vi "Dresden R2R Sputter 03.02.2018 IY24.vi"() -> ()   [LabVIEW 2009] (continued)
                                n22000 = Or(x=w22962, y=w22961) -> (x .or. y?=w22960:bool)
                                }
                                }
                                frame #1 {
                                }
                                }
                                }
                                frame #1 {
                                n22001 = local read "Semi"() -> (w22973:bool)
                                n22002 = case shown="False" w22973 {
                                frame #0 {
                                n22003 = Wait Until Next ms Multiple(millisecond multiple=u32 1000) -> ()  [unwired: 1 out]
                                n22004 = local write "Ch4_PA22"(TRUE ("PA3")) -> ()
                                }
                                frame #1 {
                                }
                                }
                                }
                                }
                              }
                              frame #1 {
                              }
                            }
                          }
                          frame #18 {
                            # "START MP"
                            n22005 = local read "Semi"() -> (w22976:bool)
                            n22006 = case shown="False" w22976 {
                              frame #0 {
                                n22007 = stacked-sequence {
                                frame #0 {
                                n22008 = local read "Semi"() -> (w22977:bool)
                                n22009 = case shown="False" w22977 {
                                frame #0 {
                                n22010 = while {
                                i -> [w22984]
                                stop <- w22978 stop-if-true
                                n22011 = Greater?(x=w22984, y=50) -> (0:w22982:bool)
                                n22012 = case shown="True" w22982 {
                                frame #0 {
                                }
                                frame #1 {
                                n22013 = local write "Semi"(TRUE ("Semi")) -> ()
                                n22014 = local write "Error Message"("Start up process  cancelled\nbecause MP4 not started.\nPlease check MP4 connections." ("Error Message")) -> ()
                                }
                                }
                                n22015 = local read "Ch4_Mp_di"() -> (w22981:bool)
                                n22016 = case shown="False" w22981 {
                                tunnel: [FALSE TRUE] -> w22980
                                frame #0 {
                                n22017 = Wait Until Next ms Multiple(millisecond multiple=u32 200) -> ()  [unwired: 1 out]
                                n22018 = local write "Ch4_Mp_do"(TRUE ("Ch1_Tp_bv_do")) -> ()
                                }
                                frame #1 {
                                }
                                }
                                n22019 = local read "Semi"() -> (w22979:bool)
                                n22020 = Or(x=w22980, y=w22979) -> (x .or. y?=w22978:bool)
                                }
                                }
                                frame #1 {
                                }
                                }
                                }
                                frame #1 {
                                n22021 = local read "Semi"() -> (w22991:bool)
                                n22022 = case shown="False" w22991 {
                                frame #0 {
                                n22023 = local write "Ch4_PA25"(TRUE ("PA3")) -> ()
                                n22024 = Wait Until Next ms Multiple(millisecond multiple=u32 1000) -> ()  [unwired: 1 out]
                                }
                                frame #1 {
                                }
                                }
                                }
                                }
                              }
                              frame #1 {
                              }
                            }
                          }
                          frame #19 {
                            # "CHECK PL-PRESSURE"
                            n22025 = local read "Semi"() -> (w22994:bool)
                            n22026 = case shown="False" w22994 {
                              frame #0 {
                                n22027 = stacked-sequence {
                                frame #0 {
                                n22028 = local read "Semi"() -> (w22995:bool)
                                n22029 = case shown="False" w22995 {
                                frame #0 {
                                n22030 = while {
                                i -> [w23004]
                                stop <- w22999 stop-if-true
                                n22031 = Greater?(x=w23004, y=1200) -> (0:w23002:bool)
                                n22032 = case shown="True" w23002 {
                                frame #0 {
                                }
                                frame #1 {
                                n22033 = local write "Semi"(TRUE ("Semi")) -> ()
                                n22034 = local write "Error Message"("Start up process was cancelled.\nPlease check Pipeline \nvacuum connections." ("Error Message")) -> ()
                                }
                                }
                                n22035 = local read "Pl_pg_press_ch4"() -> (w22998:dbl)
                                n22036 = Less?(x=w22998, y=0.9) -> (x < y?=w22996:bool)
                                n22037 = case shown="False" w22996 {
                                tunnel: [FALSE TRUE] -> w23001
                                frame #0 {
                                n22038 = Wait Until Next ms Multiple(millisecond multiple=u32 500) -> ()  [unwired: 1 out]
                                }
                                frame #1 {
                                }
                                }
                                n22039 = local read "Semi"() -> (w23000:bool)
                                n22040 = Or(x=w23001, y=w23000) -> (x .or. y?=w22999:bool)
                                }
                                }
                                frame #1 {
                                }
                                }
                                }
                                frame #1 {
                                n22041 = local read "Semi"() -> (w23010:bool)
                                n22042 = case shown="False" w23010 {
                                frame #0 {
                                n22043 = local write "Ch4_PA26"(TRUE ("PA3")) -> ()
                                n22044 = Wait Until Next ms Multiple(millisecond multiple=u32 1000) -> ()  [unwired: 1 out]
                                }
                                frame #1 {
                                }
                                }
                                }
                                }
                              }
                              frame #1 {
                              }
                            }
                          }
                          frame #20 {
                            # "START TP"
                            n22045 = local read "Semi"() -> (w23013:bool)
                            n22046 = case shown="False" w23013 {
                              frame #0 {
                                n22047 = stacked-sequence {
                                frame #0 {
                                n22048 = local read "Semi"() -> (w23014:bool)
                                n22049 = case shown="False" w23014 {
                                frame #0 {
                                n22050 = stacked-sequence {
                                frame #0 {
                                n22051 = local read "Semi"() -> (w23015:bool)
                                n22052 = case shown="False" w23015 {
                                frame #0 {
                                n22053 = local write "Tp4_auto_start"(TRUE ("Tp1_auto_start")) -> ()
                                }
                                frame #1 {
                                }
                                }
                                }
                                frame #1 {
                                n22054 = local read "Semi"() -> (w23017:bool)
                                n22055 = case shown="False" w23017 {
                                frame #0 {
                                n22056 = Wait (ms)(milliseconds to wait=u32 1000) -> ()  [unwired: 1 out]
                                }
                                frame #1 {
                                }
                                }
                                }
                                frame #2 {
                                n22057 = local read "Semi"() -> (w23019:bool)
                                n22058 = case shown="False" w23019 {
                                frame #0 {
                                n22059 = local write "Tp4_auto_start"(TRUE ("Tp1_auto_start")) -> ()
                                }
                                frame #1 {
                                }
                                }
                                }
                                }
                                }
                                frame #1 {
                                }
                                }
                                }
                                frame #1 {
                                n22060 = local read "Semi"() -> (w23021:bool)
                                n22061 = case shown="False" w23021 {
                                frame #0 {
                                n22062 = local write "Ch4_PA30"(TRUE ("PA3")) -> ()
                                n22063 = Wait Until Next ms Multiple(millisecond multiple=u32 1000) -> ()  [unwired: 1 out]
                                }
                                frame #1 {
                                }
                                }
                                }
                                }
                              }
                              frame #1 {
                              }
                            }
                          }
                          frame #21 {
                            # "CHECK CH-PRESSURE"
                            n22064 = local read "Semi"() -> (w23024:bool)
                            n22065 = case shown="False" w23024 {
                              frame #0 {
                                n22066 = stacked-sequence {
                                frame #0 {
                                n22067 = local read "Semi"() -> (w23025:bool)
                                n22068 = case shown="False" w23025 {
                                frame #0 {
                                n22069 = while {
                                i -> [w23034]
                                stop <- w23029 stop-if-true
                                n22070 = Greater?(x=w23034, y=1200) -> (0:w23032:bool)
                                n22071 = case shown="True" w23032 {
                                frame #0 {
                                }
                                frame #1 {
                                n22072 = local write "Semi"(TRUE ("Semi")) -> ()
                                n22073 = local write "Error Message"("Start up process was cancelled.\nPlease check chamber \nvacuum connections." ("Error Message")) -> ()
                                }
                                }
                                n22074 = local read "Ch4pressure"() -> (w23028:dbl)
                                n22075 = Less?(x=w23028, y=0.9) -> (x < y?=w23026:bool)
                                n22076 = case shown="False" w23026 {
                                tunnel: [FALSE TRUE] -> w23031
                                frame #0 {
                                n22077 = Wait Until Next ms Multiple(millisecond multiple=u32 500) -> ()  [unwired: 1 out]
                                }
                                frame #1 {
                                }
                                }
                                n22078 = local read "Semi"() -> (w23030:bool)
                                n22079 = Or(x=w23031, y=w23030) -> (x .or. y?=w23029:bool)
                                }
                                }
                                frame #1 {
                                }
                                }
                                }
                                frame #1 {
                                n22080 = local read "Semi"() -> (w23040:bool)
                                n22081 = case shown="False" w23040 {
                                frame #0 {
                                n22082 = local write "Ch4_PA27"(TRUE ("PA3")) -> ()
                                n22083 = Wait Until Next ms Multiple(millisecond multiple=u32 1000) -> ()  [unwired: 1 out]
                                }
                                frame #1 {
                                }
                                }
                                }
                                }
                              }
                              frame #1 {
                              }
                            }
                          }
                          frame #22 {
                            # "OPEN BG-BV"
                            n22084 = local read "Semi"() -> (w23043:bool)
                            n22085 = case shown="False" w23043 {
                              frame #0 {
                                n22086 = stacked-sequence {
                                frame #0 {
                                n22087 = local read "Semi"() -> (w23044:bool)
                                n22088 = case shown="False" w23044 {
                                frame #0 {
                                n22089 = while {
                                i -> [w23051]
                                stop <- w23046 stop-if-true
                                n22090 = Greater?(x=w23051, y=50) -> (0:w23049:bool)
                                n22091 = case shown="True" w23049 {
                                frame #0 {
                                }
                                frame #1 {
                                n22092 = local write "Semi"(TRUE ("Semi")) -> ()
                                n22093 = local write "Error Message"("Start up process  cancelled\nbecause  BG-BV not opened.\nPlease check BG-BV4 connections." ("Error Message")) -> ()
                                }
                                }
                                n22094 = local read "Ch4_Bg_bv_di"() -> (w23045:bool)
                                n22095 = case shown="False" w23045 {
                                tunnel: [FALSE TRUE] -> w23048
                                frame #0 {
                                n22096 = Wait Until Next ms Multiple(millisecond multiple=u32 200) -> ()  [unwired: 1 out]
                                n22097 = local write "Ch4_Bg_bv_do"(TRUE ("Ch1_Tp_bv_do")) -> ()
                                }
                                frame #1 {
                                }
                                }
                                n22098 = local read "Semi"() -> (w23047:bool)
                                n22099 = Or(x=w23048, y=w23047) -> (x .or. y?=w23046:bool)
                                }
                                }
                                frame #1 {
                                }
                                }
                                }
                                frame #1 {
                                n22100 = local read "Semi"() -> (w23058:bool)
                                n22101 = case shown="False" w23058 {
                                frame #0 {
                                n22102 = local write "Ch4_PA28"(TRUE ("PA3")) -> ()
                                n22103 = Wait Until Next ms Multiple(millisecond multiple=u32 1000) -> ()  [unwired: 1 out]
                                }
                                frame #1 {
                                }
                                }
                                }
                                }
                              }
                              frame #1 {
                              }
                            }
                          }
                          frame #23 {
                            # "CHECK CH-PRESSURE"
                            n22104 = local read "Semi"() -> (w23061:bool)
                            n22105 = case shown="False" w23061 {
                              frame #0 {
                                n22106 = stacked-sequence {
                                frame #0 {
                                n22107 = local read "Semi"() -> (w23062:bool)
                                n22108 = case shown="False" w23062 {
                                frame #0 {
                                n22109 = while {
                                i -> [w23071]
                                stop <- w23066 stop-if-true
                                n22110 = Greater?(x=w23071, y=600) -> (0:w23069:bool)
                                n22111 = case shown="True" w23069 {
                                frame #0 {
                                }
                                frame #1 {
                                n22112 = local write "Semi"(TRUE ("Semi")) -> ()
                                n22113 = local write "Error Message"("Start up process was cancelled.\nPlease check chamber \nvacuum connections." ("Error Message")) -> ()
                                }
                                }
                                n22114 = local read "Ch4pressure"() -> (w23065:dbl)
                                n22115 = Less?(x=w23065, y=0.9) -> (x < y?=w23063:bool)
                                n22116 = case shown="False" w23063 {
                                tunnel: [FALSE TRUE] -> w23068
                                frame #0 {
                                n22117 = Wait Until Next ms Multiple(millisecond multiple=u32 500) -> ()  [unwired: 1 out]
                                }
                                frame #1 {
                                }
                                }
                                n22118 = local read "Semi"() -> (w23067:bool)
                                n22119 = Or(x=w23068, y=w23067) -> (x .or. y?=w23066:bool)
                                }
                                }
                                frame #1 {
                                }
                                }
                                }
                                frame #1 {
                                n22120 = local read "Semi"() -> (w23077:bool)
                                n22121 = case shown="False" w23077 {
                                frame #0 {
                                n22122 = local write "Ch4_PA29"(TRUE ("PA3")) -> ()
                                n22123 = Wait Until Next ms Multiple(millisecond multiple=u32 1000) -> ()  [unwired: 1 out]
                                }
                                frame #1 {
                                }
                                }
                                }
                                }
                              }
                              frame #1 {
                              }
                            }
                          }
                          frame #24 {
                            # "START TP"
                            n22124 = local read "Semi"() -> (w23080:bool)
                            n22125 = case shown="False" w23080 {
                              frame #0 {
                                n22126 = stacked-sequence {
                                frame #0 {
                                n22127 = local read "Semi"() -> (w23081:bool)
                                n22128 = case shown="False" w23081 {
                                frame #0 {
                                n22129 = stacked-sequence {
                                frame #0 {
                                n22130 = local read "Semi"() -> (w23082:bool)
                                n22131 = case shown="False" w23082 {
                                frame #0 {
                                n22132 = local write "Tp4_auto_start"(TRUE ("Tp1_auto_start")) -> ()
                                }
                                frame #1 {
                                }
                                }
                                }
                                frame #1 {
                                n22133 = local read "Semi"() -> (w23084:bool)
                                n22134 = case shown="False" w23084 {
                                frame #0 {
                                n22135 = Wait (ms)(milliseconds to wait=u32 1000) -> ()  [unwired: 1 out]
                                }
                                frame #1 {
                                }
                                }
                                }
                                frame #2 {
                                n22136 = local read "Semi"() -> (w23086:bool)
                                n22137 = case shown="False" w23086 {
                                frame #0 {
                                n22138 = while {
                                i -> [w23092]
                                stop <- w23088 stop-if-true
                                n22139 = local read "TP4_working"() -> (w23090:bool)
                                n22140 = Greater?(x=w23092, y=120) -> (0:w23091:bool)
                                n22141 = local read "Semi"() -> (w23089:bool)
                                n22142 = Compound Arithmetic op=OR(w23089, w23090, w23091) -> (w23088:bool)
                                n22143 = Wait (ms)(milliseconds to wait=u32 500) -> ()  [unwired: 1 out]
                                }
                                }
                                frame #1 {
                                }
                                }
                                }
                                frame #3 {
                                n22144 = local read "Semi"() -> (w23094:bool)
                                n22145 = case shown="False" w23094 {
                                frame #0 {
                                n22146 = local read "TP4_working"() -> (w23095:bool)
                                n22147 = case shown="False" w23095 {
                                frame #0 {
                                n22148 = local write "Tp4_auto_start"(TRUE ("Pc_bv1_auto_open")) -> ()
                                }
                                frame #1 {
                                }
                                }
                                }
                                frame #1 {
                                }
                                }
                                }
                                frame #4 {
                                n22149 = local read "Semi"() -> (w23097:bool)
                                n22150 = case shown="False" w23097 {
                                frame #0 {
                                n22151 = local read "TP4_working"() -> (w23098:bool)
                                n22152 = case shown="False" w23098 {
                                frame #0 {
                                n22153 = Wait (ms)(milliseconds to wait=u32 1000) -> ()  [unwired: 1 out]
                                }
                                frame #1 {
                                }
                                }
                                }
                                frame #1 {
                                }
                                }
                                }
                                frame #5 {
                                n22154 = local read "Semi"() -> (w23100:bool)
                                n22155 = case shown="False" w23100 {
                                frame #0 {
                                n22156 = while {
                                i -> [w23106]
                                stop <- w23102 stop-if-true
                                n22157 = local read "TP4_working"() -> (w23104:bool)
                                n22158 = Greater?(x=w23106, y=120) -> (0:w23105:bool)
                                n22159 = local read "Semi"() -> (w23103:bool)
                                n22160 = Compound Arithmetic op=OR(w23103, w23104, w23105) -> (w23102:bool)
                                n22161 = Wait (ms)(milliseconds to wait=u32 500) -> ()  [unwired: 1 out]
                                }
                                }
                                frame #1 {
                                }
                                }
                                }
                                frame #6 {
                                n22162 = local read "Semi"() -> (w23108:bool)
                                n22163 = case shown="False" w23108 {
                                frame #0 {
                                n22164 = local read "TP4_working"() -> (w23109:bool)
                                n22165 = case shown="False" w23109 {
                                frame #0 {
                                n22166 = local write "Error Message"("Start up process  cancelled\nbecause  TP not started.\nPlease check TP4 connections." ("Error Message")) -> ()
                                n22167 = Wait (ms)(milliseconds to wait=u32 1000) -> ()  [unwired: 1 out]
                                }
                                frame #1 {
                                }
                                }
                                }
                                frame #1 {
                                }
                                }
                                }
                                }
                                }
                                frame #1 {
                                }
                                }
                                }
                                frame #1 {
                                n22168 = local read "Semi"() -> (w23112:bool)
                                n22169 = case shown="False" w23112 {
                                frame #0 {
                                n22170 = local write "Ch4_PA30"(TRUE ("PA3")) -> ()
                                n22171 = Wait Until Next ms Multiple(millisecond multiple=u32 1000) -> ()  [unwired: 1 out]
                                }
                                frame #1 {
                                }
                                }
                                }
                                }
                              }
                              frame #1 {
                              }
                            }
                          }
                          frame #25 {
                            # "CHECK CH-PRESSURE"
                            n22172 = local read "Semi"() -> (w23115:bool)
                            n22173 = case shown="False" w23115 {
                              frame #0 {
                                n22174 = stacked-sequence {
                                frame #0 {
                                n22175 = local read "Semi"() -> (w23116:bool)
                                n22176 = case shown="False" w23116 {
                                frame #0 {
                                n22177 = while {
                                i -> [w23125]
                                stop <- w23120 stop-if-true
                                n22178 = Greater?(x=w23125, y=240) -> (0:w23123:bool)
                                n22179 = case shown="True" w23123 {
                                frame #0 {
                                }
                                frame #1 {
                                n22180 = local write "Semi"(TRUE ("Semi")) -> ()
                                n22181 = local write "Error Message"("Start up process was cancelled.\nPlease check chamber \nvacuum connections." ("Error Message")) -> ()
                                }
                                }
                                n22182 = local read "Ch4pressure"() -> (w23119:dbl)
                                n22183 = Less?(x=w23119, y=0.9) -> (x < y?=w23117:bool)
                                n22184 = case shown="False" w23117 {
                                tunnel: [FALSE TRUE] -> w23122
                                frame #0 {
                                n22185 = Wait Until Next ms Multiple(millisecond multiple=u32 500) -> ()  [unwired: 1 out]
                                }
                                frame #1 {
                                }
                                }
                                n22186 = local read "Semi"() -> (w23121:bool)
                                n22187 = Or(x=w23122, y=w23121) -> (x .or. y?=w23120:bool)
                                }
                                }
                                frame #1 {
                                }
                                }
                                }
                                frame #1 {
                                n22188 = local read "Semi"() -> (w23131:bool)
                                n22189 = case shown="False" w23131 {
                                frame #0 {
                                n22190 = local write "Ch4_PA31"(TRUE ("PA3")) -> ()
                                n22191 = Wait Until Next ms Multiple(millisecond multiple=u32 1000) -> ()  [unwired: 1 out]
                                }
                                frame #1 {
                                }
                                }
                                }
                                }
                              }
                              frame #1 {
                              }
                            }
                          }
                        }
                      }
                      frame #1 {
                      }
                    }
                  }
                }
              }
              frame #1 {
              }
            }
          }
          frame #2 {
            # "ROUTINE CHECK"
            n22192 = local read "Semi"() -> (w23134:bool)
            n22193 = case shown="False" w23134 {
              frame #0 {
                n22194 = stacked-sequence {
                  frame #0 {
                    n22195 = local read "Semi"() -> (w23135:bool)
                    n22196 = case shown="False" w23135 {
                      frame #0 {
                        n22197 = stacked-sequence {
                          frame #0 {
                            n22198 = local read "Semi"() -> (w23136:bool)
                            n22199 = case shown="False" w23136 {
                              frame #0 {
                                n22200 = while {
                                i -> [w23145]
                                stop <- w23140 stop-if-true
                                n22201 = Greater?(x=w23145, y=400) -> (0:w23143:bool)
                                n22202 = case shown="True" w23143 {
                                frame #0 {
                                }
                                frame #1 {
                                n22203 = local write "Error Message"("Start up process was cancelled.\nPlease check Chamber \nvacuum connections." ("Error Message")) -> ()
                                n22204 = local write "Semi"(TRUE ("Semi")) -> ()
                                }
                                }
                                n22205 = local read "Ch4pressure"() -> (w23137:dbl)
                                n22206 = Less?(x=w23137, y=0.01) -> (x < y?=w23138:bool)
                                n22207 = case shown="False" w23138 {
                                tunnel: [TRUE FALSE] -> w23142
                                frame #0 {
                                }
                                frame #1 {
                                n22208 = Wait Until Next ms Multiple(millisecond multiple=u32 500) -> ()  [unwired: 1 out]
                                }
                                }
                                n22209 = local read "Semi"() -> (w23141:bool)
                                n22210 = Or(x=w23142, y=w23141) -> (x .or. y?=w23140:bool)
                                }
                              }
                              frame #1 {
                              }
                            }
                          }
                          frame #1 {
                            n22211 = local read "Semi"() -> (w23151:bool)
                            n22212 = case shown="False" w23151 {
                              frame #0 {
                                n22213 = Wait Until Next ms Multiple(millisecond multiple=u32 1000) -> ()  [unwired: 1 out]
                              }
                              frame #1 {
                              }
                            }
                          }
                        }
                      }
                      frame #1 {
                      }
                    }
                  }
                  frame #1 {
                    n22214 = local read "Semi"() -> (w23153:bool)
                    n22215 = case shown="False" w23153 {
                      frame #0 {
                        n22216 = stacked-sequence {
                          frame #0 {
                            n22217 = local read "Semi"() -> (w23154:bool)
                            n22218 = case shown="False" w23154 {
                              frame #0 {
                                n22219 = while {
                                i -> [w23161]
                                stop <- w23155 stop-if-true
                                n22220 = Greater?(x=w23161, y=90) -> (0:w23159:bool)
                                n22221 = case shown="True" w23159 {
                                frame #0 {
                                }
                                frame #1 {
                                n22222 = local write "Semi"(TRUE ("Semi")) -> ()
                                n22223 = local write "Error Message"("Start up process  cancelled\nbecause  CC not opened.\nPlease check CH4-CC connections." ("Error Message")) -> ()
                                }
                                }
                                n22224 = local read "Ch4_Cc_on_off_di"() -> (w23158:bool)
                                n22225 = case shown="False" w23158 {
                                tunnel: [TRUE FALSE] -> w23157
                                frame #0 {
                                }
                                frame #1 {
                                n22226 = Wait Until Next ms Multiple(millisecond multiple=u32 200) -> ()  [unwired: 1 out]
                                n22227 = local write "Ch4_Cc_on_off_do"(TRUE ("Ch1_Tp_bv_do")) -> ()
                                }
                                }
                                n22228 = local read "Semi"() -> (w23156:bool)
                                n22229 = Or(x=w23157, y=w23156) -> (x .or. y?=w23155:bool)
                                }
                              }
                              frame #1 {
                              }
                            }
                          }
                          frame #1 {
                            n22230 = local read "Semi"() -> (w23168:bool)
                            n22231 = case shown="False" w23168 {
                              frame #0 {
                                n22232 = while {
                                i -> [w23172]
                                stop <- w23169 stop-if-true
                                n22233 = Greater Or Equal?(x=w23172, y=150) -> (x >= y?=w23170:bool)
                                n22234 = Wait (ms)(milliseconds to wait=u32 200) -> ()  [unwired: 1 out]
                                n22235 = local read "Semi"() -> (w23174:bool)
                                n22236 = Compound Arithmetic op=OR(w23170, w23174) -> (w23169:bool)
                                }
                              }
                              frame #1 {
                              }
                            }
                          }
                          frame #2 {
                            n22237 = local read "Semi"() -> (w23175:bool)
                            n22238 = case shown="False" w23175 {
                              frame #0 {
                                n22239 = local write "Ch4_PA32"(TRUE ("P1")) -> ()
                                n22240 = local write "Ch4_PV19"(TRUE ("P1")) -> ()
                                n22241 = Wait Until Next ms Multiple(millisecond multiple=u32 2000) -> ()  [unwired: 1 out]
                              }
                              frame #1 {
                              }
                            }
                          }
                        }
                      }
                      frame #1 {
                      }
                    }
                  }
                  frame #2 {
                    n22242 = local read "Semi"() -> (w23179:bool)
                    n22243 = case shown="False" w23179 {
                      frame #0 {
                        n22244 = stacked-sequence {
                          frame #0 {
                            n22245 = local read "Semi"() -> (w23180:bool)
                            n22246 = case shown="False" w23180 {
                              frame #0 {
                                n22247 = while {
                                i -> [w23187]
                                stop <- w23181 stop-if-true
                                n22248 = Greater?(x=w23187, y=90) -> (0:w23185:bool)
                                n22249 = case shown="True" w23185 {
                                frame #0 {
                                }
                                frame #1 {
                                n22250 = local write "Semi"(TRUE ("Semi")) -> ()
                                n22251 = local write "Error Message"("Start up process  cancelled\nbecause  CH4-Trns-GV-BP\n not opened.\nPlease check CH4-Trns-GV-BP\nconnections." ("Error Message")) -> ()
                                }
                                }
                                n22252 = local read "Ch4_Trns_gv_bp_di"() -> (w23184:bool)
                                n22253 = case shown="True" w23184 {
                                tunnel: [FALSE TRUE] -> w23183
                                frame #0 {
                                n22254 = Wait Until Next ms Multiple(millisecond multiple=u32 200) -> ()  [unwired: 1 out]
                                n22255 = local write "Ch4_Trns_gv_bp_do"(FALSE ("Ch1_Tp_bv_do")) -> ()
                                }
                                frame #1 {
                                }
                                }
                                n22256 = local read "Semi"() -> (w23182:bool)
                                n22257 = Or(x=w23183, y=w23182) -> (x .or. y?=w23181:bool)
                                }
                              }
                              frame #1 {
                              }
                            }
                          }
                          frame #1 {
                            n22258 = local read "Semi"() -> (w23194:bool)
                            n22259 = case shown="False" w23194 {
                              frame #0 {
                                n22260 = local write "Ch4_PV20"(TRUE ("P1")) -> ()
                                n22261 = local write "Ch4_PA33"(TRUE ("P1")) -> ()
                                n22262 = Wait Until Next ms Multiple(millisecond multiple=u32 2000) -> ()  [unwired: 1 out]
                              }
                              frame #1 {
                              }
                            }
                          }
                        }
                      }
                      frame #1 {
                      }
                    }
                  }
                  frame #3 {
                    n22263 = local read "Semi"() -> (w23198:bool)
                    n22264 = case shown="False" w23198 {
                      frame #0 {
                        n22265 = stacked-sequence {
                          frame #0 {
                            n22266 = local read "Semi"() -> (w23199:bool)
                            n22267 = case shown="False" w23199 {
                              frame #0 {
                                n22268 = while {
                                i -> [w23208]
                                stop <- w23203 stop-if-true
                                n22269 = local read "Target_time_ch4"() -> (w23202:dbl)
                                n22270 = Multiply(x=w23202, y=7200) -> (x*y=w23200:dbl)
                                n22271 = Greater?(x=w23208, y=w23200) -> (0:w23207:bool)
                                n22272 = case shown="True" w23207 {
                                frame #0 {
                                }
                                frame #1 {
                                n22273 = local write "Semi"(TRUE ("Semi")) -> ()
                                }
                                }
                                n22274 = local read "Semi"() -> (w23206:bool)
                                n22275 = case shown="False" w23206 {
                                tunnel: [TRUE w23213] -> w23205
                                frame #0 {
                                }
                                frame #1 {
                                n22276 = local read "Target Pressure_ch4"() -> (w23212:dbl)
                                n22277 = local read "Ch4_pressure2"() -> (w23211:dbl)
                                n22278 = Less Or Equal?(x=w23212, y=w23211) -> (x <= y?=w23210:bool)
                                n22279 = case shown="True" w23210 {
                                tunnel: [TRUE FALSE] -> w23213
                                frame #0 {
                                }
                                frame #1 {
                                n22280 = Wait Until Next ms Multiple(millisecond multiple=u32 750) -> ()  [unwired: 1 out]
                                }
                                }
                                }
                                }
                                n22281 = local read "Semi"() -> (w23204:bool)
                                n22282 = Or(x=w23205, y=w23204) -> (x .or. y?=w23203:bool)
                                }
                              }
                              frame #1 {
                              }
                            }
                          }
                          frame #1 {
                            n22283 = local read "Semi"() -> (w23218:bool)
                            n22284 = case shown="False" w23218 {
                              frame #0 {
                                n22285 = Wait (ms)(milliseconds to wait=u32 1000) -> ()  [unwired: 1 out]
                              }
                              frame #1 {
                              }
                            }
                          }
                          frame #2 {
                            n22286 = local read "Semi"() -> (w23220:bool)
                            n22287 = case shown="False" w23220 {
                              frame #0 {
                                n22288 = local write "Ch4_PV21"(TRUE ("P1")) -> ()
                                n22289 = local write "Ch4_PA34"(TRUE ("P1")) -> ()
                                n22290 = Wait Until Next ms Multiple(millisecond multiple=u32 1000) -> ()  [unwired: 1 out]
                              }
                              frame #1 {
                              }
                            }
                          }
                        }
                      }
                      frame #1 {
                      }
                    }
                  }
                }
              }
              frame #1 {